vi "Panel.vi"() -> ()   [LabVIEW 2020]
uses:
  Mete.ctl
  R.ctl
  P.ctl
  N.ctl
  D.ctl
  Odo Velocity.ctl
  Gas.ctl
panel:
  in  "Slide 2":T1
  out "Km/h":T2 scale=0.0..250.0
  in  "stop":bool
  in  "Slide":u32(slide) max=900 scale=0.0..999.0
  in  "Boolean 8":bool
  in  "Boolean 7":bool
  in  "Boolean 6":bool
  in  "Boolean 5":bool
  out "Boolean 4":T3
  out "Boolean 3":T4
  out "Boolean 2":T5
  out "Boolean":T6
  out "Gauge":T7 scale=0.0..650.0
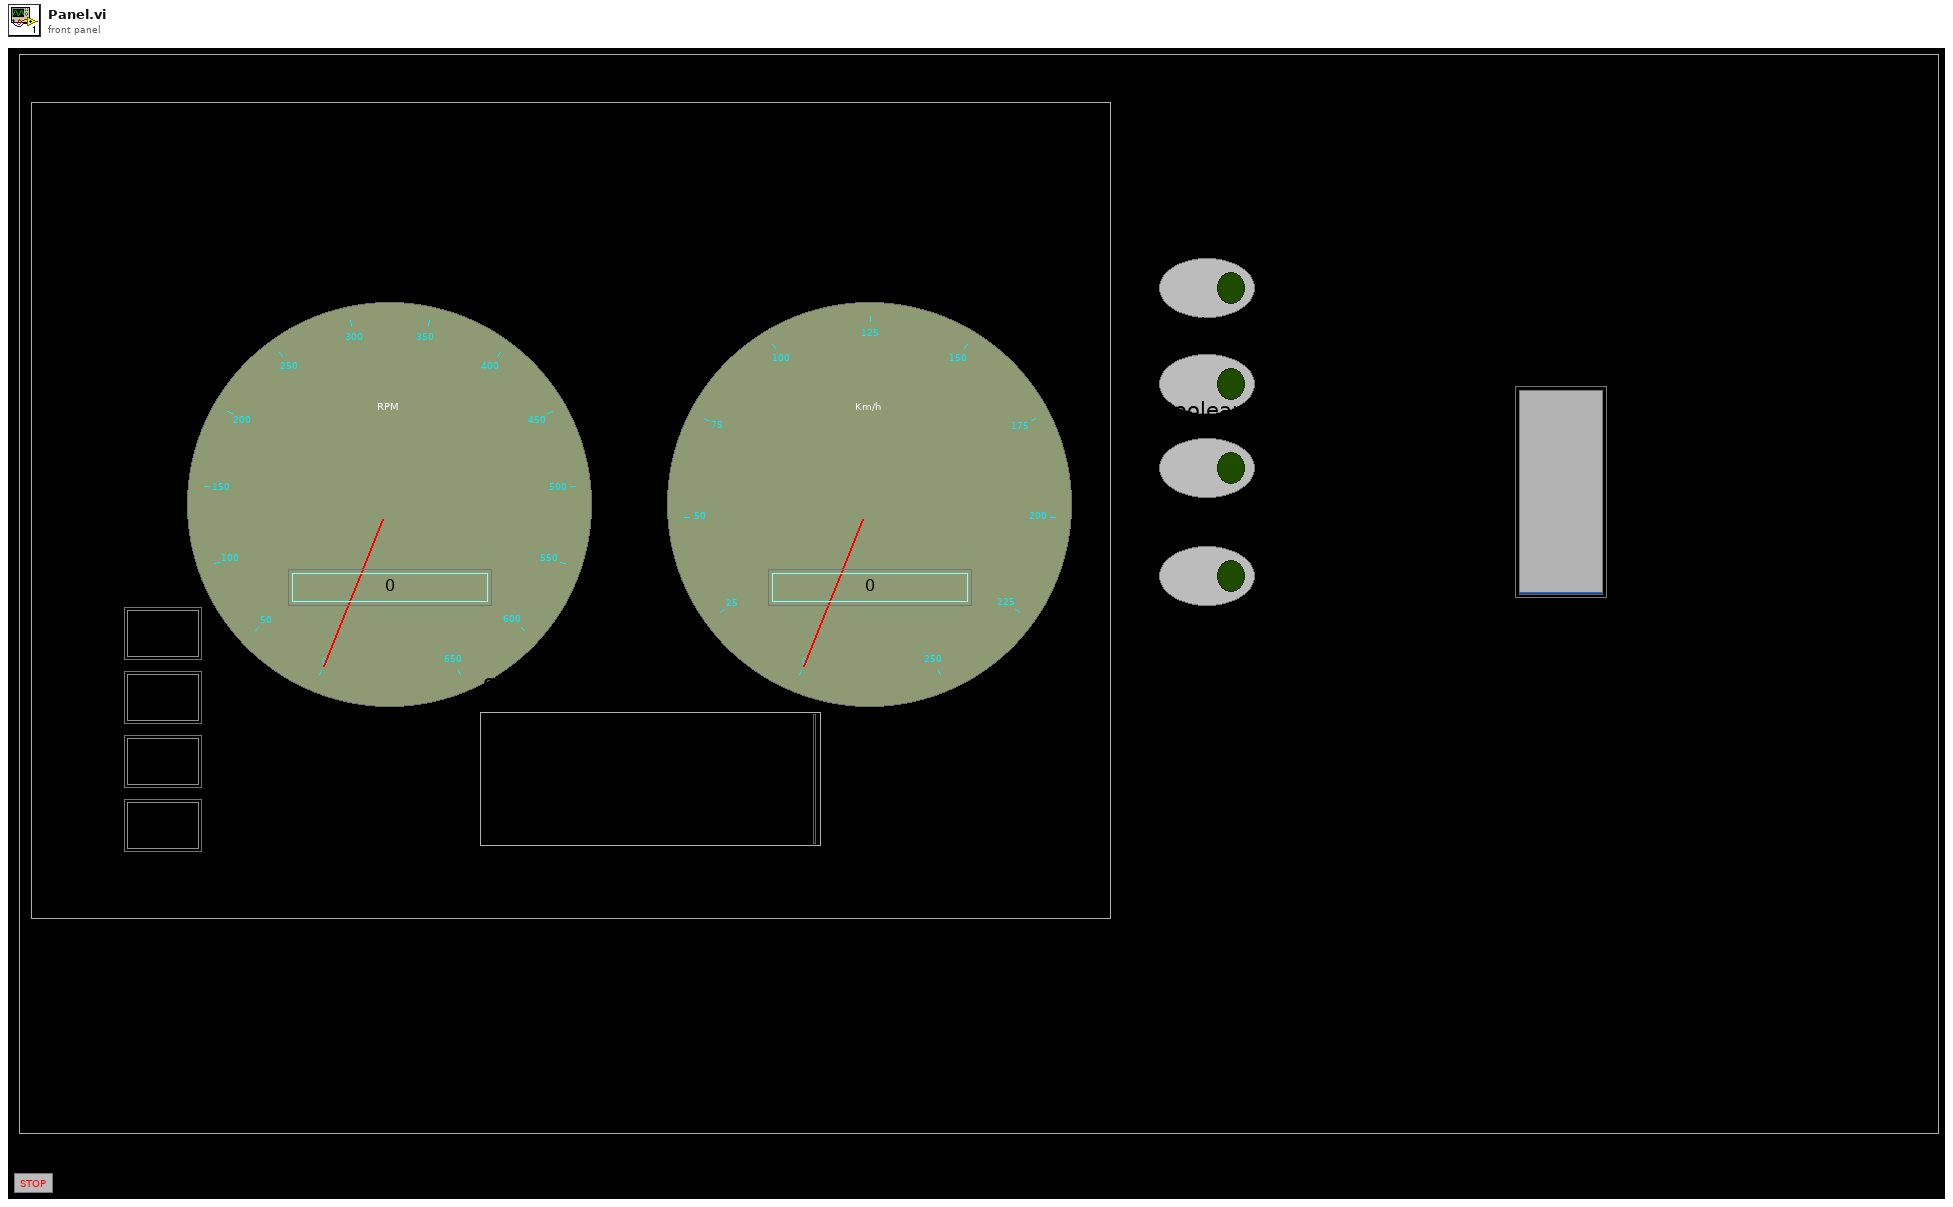
[diagram p1: front panel]
types:
  T1 = typedef "Gas.ctl" = dbl
  T2 = typedef "Odo Velocity.ctl" = u16
  T3 = typedef "D.ctl" = bool
  T4 = typedef "N.ctl" = bool
  T5 = typedef "P.ctl" = bool
  T6 = typedef "R.ctl" = bool
  T7 = typedef "Mete.ctl" = u16
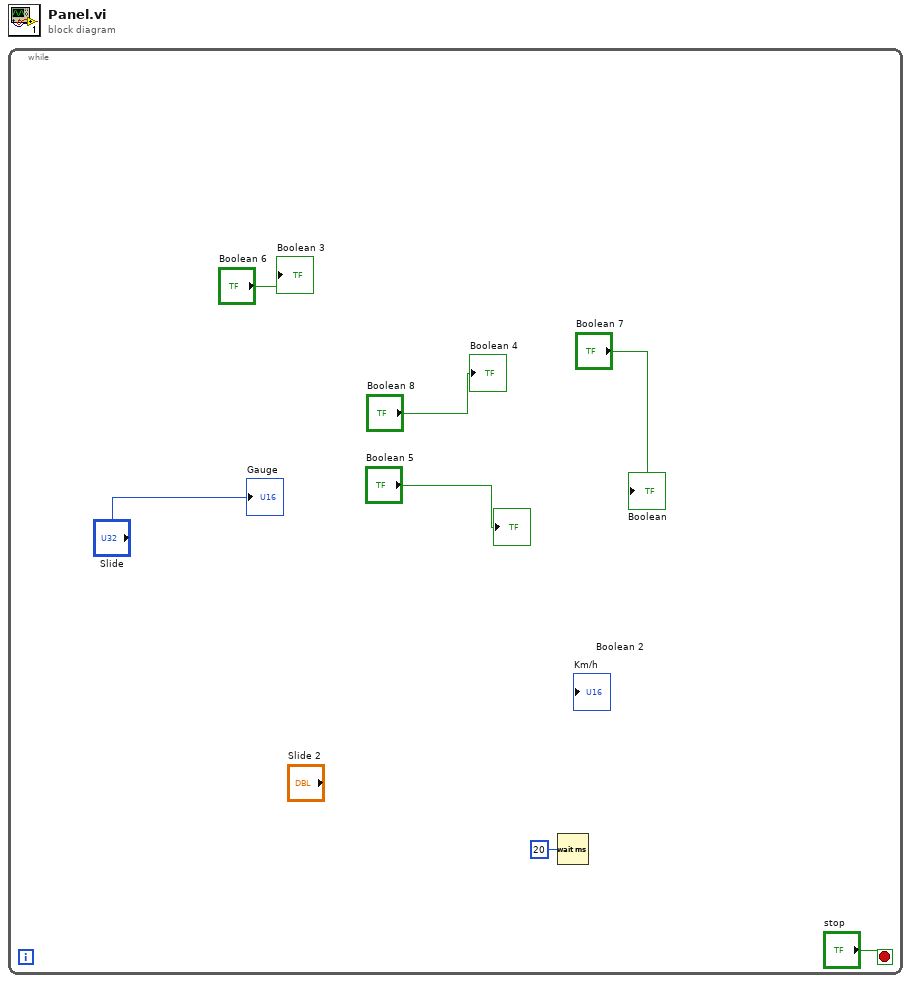
[diagram p0: block diagram]
diagram:
  n1 = while {
    stop <- "stop" stop-if-true
    n2 = Wait (ms)(milliseconds to wait=u32 20) -> ()  [unwired: 1 out]
    "Gauge" <- "Slide"
    "Boolean 2" <- "Boolean 5"
    "Boolean 3" <- "Boolean 6"
    "Boolean" <- "Boolean 7"
    "Boolean 4" <- "Boolean 8"
  }
